vi "CRYO_MASTER_FULL_RUN3.vi"() -> ()   [LabVIEW 2017] (continued)
  in  "CONTROL KIKUSUI?":bool=TRUE
  in  "OUTPUT\n(PWR)":bool
  in  "Set Current (mA)\n (PWR)":dbl=4.0 min=4.0 max=20.0 format="%_3g"
  out "RUN Identifier 5":string="20210209_084357_RUNIII" caption="RUN Identifier"
  in  "DMMsConfig":T11(array[cluster])=[{"Label"="I_H1", "Active?"=TRUE, "VISA resource name"="USB0::0x1334::0x0204::262800066::INSTR", "Device"=enum."ADCMT7351", "Measurement"=enum."DC Currents", "FileFormat"="%.4e"}, {"Label"="V_H1", "Active?"=TRUE, "VISA resource name"="USB0::0x1334::0x0204::262800451::INSTR", "Device"=enum."ADCMT7351", "Measurement"=enum."DC Volts", "FileFormat"="%.4e"}, {"Label"="I_H2", "Active?"=TRUE, "VISA resource name"="GPIB0::23::INSTR", "Device"=enum."ADCMT7451", "Measurement"=enum."DC Currents", "FileFormat"="%.4e"}, {"Label"="V_H2", "Active?"=TRUE, "VISA resource name"="GPIB0::22::INSTR", "Device"=enum."Agilent34401A", "Measurement"=enum."DC Volts", "FileFormat"="%.4e"}, {"Label"="I_H4", "Active?"=TRUE, "VISA resource name"="GPIB0::21::INSTR", "Device"=enum."Agilent34401A", "Measurement"=enum."DC Currents", "FileFormat"="%.4e"}, {"Label"="V_H4", "Active?"=TRUE, "VISA resource name"="GPIB0::25::INSTR", "Device"=enum."Agilent34401A", "Measurement"=enum."DC Volts", "FileFormat"="%.4e"}]
  out "ƒ¢T=T_2 -T_1":dbl=-101388.71309149737
  out "Graph DMMs 3":T4(graph)=[{"TimeArray"=[timestamp(3695672642.6155486 s since 1904-01-01)], "DataArray"=[-2.68e-05]}, {"TimeArray"=[timestamp(3695672642.6155486 s since 1904-01-01)], "DataArray"=[-0.0014684]}, {"TimeArray"=[timestamp(3695672642.6155486 s since 1904-01-01)], "DataArray"=[-1.232e-05]}, {"TimeArray"=[timestamp(3695672642.6155486 s since 1904-01-01)], "DataArray"=[2.8262e-06]}, {"TimeArray"=[timestamp(3695672642.6155486 s since 1904-01-01)], "DataArray"=[3.71392e-06]}, {"TimeArray"=[timestamp(3695672642.6155486 s since 1904-01-01)], "DataArray"=[0.000182]}, {"TimeArray"=[timestamp(3695672642.6155486 s since 1904-01-01)], "DataArray"=[101407.09548804205]}, {"TimeArray"=[timestamp(3695672642.6155486 s since 1904-01-01)], "DataArray"=[-0.36185606613019977]}, {"TimeArray"=[timestamp(3695672642.6155486 s since 1904-01-01)], "DataArray"=[-3.0973798990583647]}, {"TimeArray"=[timestamp(3695672642.6155486 s since 1904-01-01)], "DataArray"=[18.382396544680894]}, {"TimeArray"=[timestamp(3695672642.6155486 s since 1904-01-01)], "DataArray"=[-48.20456535494683]}, {"TimeArray"=[timestamp(3695672642.6155486 s since 1904-01-01)], "DataArray"=[167.919]}, {"TimeArray"=[timestamp(3695672642.6155486 s since 1904-01-01)], "DataArray"=[163.1]}, {"TimeArray"=[timestamp(3695672642.6155486 s since 1904-01-01)], "DataArray"=[162.659]}, {"TimeArray"=[timestamp(3695672642.6155486 s since 1904-01-01)], "DataArray"=[160.848]}] caption="XY Graph"
  out "Q = I *V":dbl=3.935312e-08
  in  "index I":i64
  in  "index V":i64=1
  out "VariableSources":T12(array[ring])=[enum."USB6210", enum."USB6218AI", enum."USB6218AI", enum."USB6218AI", enum."USB6210", enum."LSI336", enum."LSI336", enum."LSI336", enum."LSI336"]
  in  "DMMsConfig (variables)":T13(array[cluster])=[{"Label"="P_3Hepot", "Active?"=TRUE, "Source"=enum."USB6210", "SourceLabel"="P_3Hepot", "FileFormat"="%6.4e"}, {"Label"="F_1", "Active?"=TRUE, "Source"=enum."USB6218AI", "SourceLabel"="F_1", "FileFormat"="%3.4f"}, {"Label"="F_4", "Active?"=TRUE, "Source"=enum."USB6218AI", "SourceLabel"="F_4", "FileFormat"="%3.4f"}, {"Label"="F_5", "Active?"=TRUE, "Source"=enum."USB6218AI", "SourceLabel"="F_5", "FileFormat"="%3.4f"}, {"Label"="DP_HEX4", "Active?"=TRUE, "Source"=enum."USB6210", "SourceLabel"="DP_HEX4", "FileFormat"="%4.3e"}, {"Label"="T3He6-1", "Active?"=TRUE, "Source"=enum."LSI336", "SourceLabel"="T3He6-1", "FileFormat"="%3.4f"}, {"Label"="T3He6-2", "Active?"=TRUE, "Source"=enum."LSI336", "SourceLabel"="T3He6-2", "FileFormat"="%3.4f"}, {"Label"="T3He7-1", "Active?"=TRUE, "Source"=enum."LSI336", "SourceLabel"="T3He7-1", "FileFormat"="%3.4f"}, {"Label"="T3He7-2", "Active?"=TRUE, "Source"=enum."LSI336", "SourceLabel"="T3He7-2", "FileFormat"="%3.4f"}]
  in  "Measure DMMs?":bool=TRUE
  out "DMMsLabels":string[](array[string])=["I_H1", "V_H1", "I_H2", "V_H2", "I_H4", "V_H4", "P_3Hepot", "F_1", "F_4", "F_5", "DP_HEX4", "T3He6-1", "T3He6-2", "T3He7-1", "T3He7-2"]
  out "Active?":bool[](array[boolean])=[TRUE, TRUE, TRUE, TRUE, TRUE, TRUE, TRUE, TRUE, TRUE, TRUE, TRUE, TRUE, TRUE, TRUE, TRUE]
  out "DMM LastMeasurements":dbl[](array[numeric])=[-2.68e-05, -0.0014684, -1.232e-05, 2.8262e-06, 3.71392e-06, 0.000182, 101407.09548804205, -0.36185606613019977, -3.0973798990583647, 18.382396544680894, -48.20456535494683, 167.919, 163.1, 162.659, 160.848]
  out "Graph DMMs 2":T4(graph)=[{"TimeArray"=[timestamp(3695672642.6155486 s since 1904-01-01)], "DataArray"=[-2.68e-05]}, {"TimeArray"=[timestamp(3695672642.6155486 s since 1904-01-01)], "DataArray"=[-0.0014684]}, {"TimeArray"=[timestamp(3695672642.6155486 s since 1904-01-01)], "DataArray"=[-1.232e-05]}, {"TimeArray"=[timestamp(3695672642.6155486 s since 1904-01-01)], "DataArray"=[2.8262e-06]}, {"TimeArray"=[timestamp(3695672642.6155486 s since 1904-01-01)], "DataArray"=[3.71392e-06]}, {"TimeArray"=[timestamp(3695672642.6155486 s since 1904-01-01)], "DataArray"=[0.000182]}, {"TimeArray"=[timestamp(3695672642.6155486 s since 1904-01-01)], "DataArray"=[101407.09548804205]}, {"TimeArray"=[timestamp(3695672642.6155486 s since 1904-01-01)], "DataArray"=[-0.36185606613019977]}, {"TimeArray"=[timestamp(3695672642.6155486 s since 1904-01-01)], "DataArray"=[-3.0973798990583647]}, {"TimeArray"=[timestamp(3695672642.6155486 s since 1904-01-01)], "DataArray"=[18.382396544680894]}, {"TimeArray"=[timestamp(3695672642.6155486 s since 1904-01-01)], "DataArray"=[-48.20456535494683]}, {"TimeArray"=[timestamp(3695672642.6155486 s since 1904-01-01)], "DataArray"=[167.919]}, {"TimeArray"=[timestamp(3695672642.6155486 s since 1904-01-01)], "DataArray"=[163.1]}, {"TimeArray"=[timestamp(3695672642.6155486 s since 1904-01-01)], "DataArray"=[162.659]}, {"TimeArray"=[timestamp(3695672642.6155486 s since 1904-01-01)], "DataArray"=[160.848]}] caption="XY Graph"
  out "DMMFileName":string="20210209_084357_RUNIII_DMMs_20210209_084357.csv"
  out "error out (DMMs)":errorcluster
  out "cycle # (DMMs)":i32=1
  in  "Measurement Interval DMMs (ms)":i64=500
  in  "InstName DMMs":string="DMMs"
  in  "Initialize (DMMs)":bool
  out "Graph DMMs 1":T4(graph)=[{"TimeArray"=[timestamp(3695672642.6155486 s since 1904-01-01)], "DataArray"=[-2.68e-05]}, {"TimeArray"=[timestamp(3695672642.6155486 s since 1904-01-01)], "DataArray"=[-0.0014684]}, {"TimeArray"=[timestamp(3695672642.6155486 s since 1904-01-01)], "DataArray"=[-1.232e-05]}, {"TimeArray"=[timestamp(3695672642.6155486 s since 1904-01-01)], "DataArray"=[2.8262e-06]}, {"TimeArray"=[timestamp(3695672642.6155486 s since 1904-01-01)], "DataArray"=[3.71392e-06]}, {"TimeArray"=[timestamp(3695672642.6155486 s since 1904-01-01)], "DataArray"=[0.000182]}, {"TimeArray"=[timestamp(3695672642.6155486 s since 1904-01-01)], "DataArray"=[101407.09548804205]}, {"TimeArray"=[timestamp(3695672642.6155486 s since 1904-01-01)], "DataArray"=[-0.36185606613019977]}, {"TimeArray"=[timestamp(3695672642.6155486 s since 1904-01-01)], "DataArray"=[-3.0973798990583647]}, {"TimeArray"=[timestamp(3695672642.6155486 s since 1904-01-01)], "DataArray"=[18.382396544680894]}, {"TimeArray"=[timestamp(3695672642.6155486 s since 1904-01-01)], "DataArray"=[-48.20456535494683]}, {"TimeArray"=[timestamp(3695672642.6155486 s since 1904-01-01)], "DataArray"=[167.919]}, {"TimeArray"=[timestamp(3695672642.6155486 s since 1904-01-01)], "DataArray"=[163.1]}, {"TimeArray"=[timestamp(3695672642.6155486 s since 1904-01-01)], "DataArray"=[162.659]}, {"TimeArray"=[timestamp(3695672642.6155486 s since 1904-01-01)], "DataArray"=[160.848]}] caption="XY Graph"
  out "error out (DMM graphs)":errorcluster
  in  "Sample #":i32=5
  in  "index T_ 1":i64=6
  in  "index T_2":i64=9
  out "error out (DMMs) 2":errorcluster
  out "P_HEX7OUT":dbl=101021.4665932051 format="%_4e"
  out "P (HEX7 out)":dbl=101021.4665932051 format="%_4e"
  out "DP HEX5":dbl=-4.397643774686294 format="%_4e"
  out "DP_HEX5":dbl=-4.397643774686294 format="%_4e"
  in  "Diff pressure HEX5":string="DP_HEX5"
  out "3He pot level":dbl=7.365405585846229 format="%_4f"
  in  "3He pot":string="L1"
  out "He level (3He)":dbl(slide)=7.365405585846229 scale=0.0..100.0
  out "He level (1K) b":dbl(slide)=-0.047872817403439266 scale=0.0..100.0
  out "He level (1K)":dbl(slide)=0.13428935722636412 scale=0.0..100.0
  out "He level (4K)":dbl(slide)=-0.023540685641880416 scale=0.0..100.0
  out "1K pot(b1)":dbl=-0.047872817403439266 format="%_4f"
  in  "1K pot (b)":string="L2-2"
  in  "1K pot level":string="L2-1"
  out "L(1K) (a1)":dbl=0.13428935722636412 format="%_4f"
  in  "SensorLocation 2":T14(ring)=enum."T3He5"
  out "Temperature 2":dbl=167.912
  out "DP HEX4":dbl=-47.57146989712546 format="%_4e"
  in  "Diff pressure HEX4":string="DP_HEX4"
  out "V2":bool
  out "V1":bool=TRUE
  out "F5 (1K pump ex.)":dbl=17.202044578830606 format="%_4f"
  out "F4 (3He in to HEX7)":dbl=-7.769469766427424 format="%_3f"
  out "F3 (4He rtn flw via HEX7)":dbl=2.98269711881182 format="%_4f"
  out "F1 (3He pump exhaust) flow":dbl=-5.195052785009831 format="%_4f"
  out "P (Dewar)":dbl=102950.69349153554 format="%_4e"
  out "P (1K pot)":dbl=101443.04292994068 format="%_4e"
  out "P (3He pot)":dbl=101551.76197190638 format="%_4e"
  out "P (shield return)":dbl=101480.26148830613 format="%_4e"
  out "P (3He IN)":dbl=100240.36414180837 format="%_4e"
  out "P (4K reservoir)":dbl=97813.1918911886 format="%_4e"
  out "P (insulation)":dbl=18.32747458588863 format="%_4e"
  in  "1Kpot pump exhaust flow":string="F_5"
  out "F_5":dbl=17.202044578830606 format="%_4f"
  in  "3He incoming flow into HEX7":string="F_4"
  out "F_4":dbl=-7.769469766427424 format="%_4f"
  out "F_3":dbl=2.98269711881182 format="%_4f"
  in  "4He return flow from HEX7":string="F_3"
  out "F_2":dbl=0.20377377393752083 format="%_4f"
  in  "Shield flow":string="F_2"
  out "P_SldRTN":dbl=101480.26148830613 format="%_4e"
  in  "3He pot pressure":string="P_3Hepot"
  out "P_3Hepot":dbl=101551.76197190638 format="%_4e"
  in  "Shield return press.":string="P_SldRTN"
  out "F_1":dbl=-5.195052785009831 format="%_4f"
  in  "3He pump exhaust flow":string="F_1"
  out "P_Dewar":dbl=102950.69349153554 format="%_4e"
  in  "Dewar pressure":string="P_Dewar"
  out "P_1Kpot":dbl=101443.04292994068 format="%_4e"
  in  "1Kpot pressure":string="P_1Kpot"
  out "P_3HeIN":dbl=100240.36414180837 format="%_4e"
  in  "3He inlet pressure":string="P_3HeIN"
  in  "4K reservoir pressure":string="P_4Kres"
  out "P_4Kres":dbl=97813.1918911886 format="%_4e"
  out "P_ins":dbl=18.32747458588863 format="%_4e"
  in  "Insulation vacuum":string="P_ins"
  out "T3He7-1/6-2 (3He pot) 2":dbl=159.065 format="%_4f"
  out "T3He7-1/7-2 (HEX1)":dbl=160.911 format="%_4f"
  out "T3He6-1/6-2 (3He pot) 2":dbl=161.329 format="%_4f"
  out "T3He6-1/6-2 (HEX1)":dbl=166.258 format="%_4f"
  out "T1K3-1/3-2 (1K pot) 2":dbl=116.203 format="%_4f"
  out "T1K3-1/3-2 (1K pot)":dbl=116.239 format="%_4f"
  out "T4He1 (4K reservoir )":dbl=127.38 format="%_4f"
  out "Temperature 1":dbl=206.95
  in  "SensorLocation 1":T14(ring)=enum."TTH2"
  out "TIP7":dbl format="%_4g"
  out "T3He6-2":dbl=161.329 format="%_4g"
  out "T3He7-2":dbl=159.065 format="%_4g"
  out "T3He6-1":dbl=166.258 format="%_4g"
  out "T3He4":dbl=154.09 format="%_4g"
  out "T3He7-1":dbl=160.911 format="%_4g"
  out "T3He8":dbl=127.318 format="%_4g"
  out "T3He5":dbl=167.912 format="%_4g"
  out "T1K3-2":dbl=116.203 format="%_4g"
  out "T1K3-1":dbl=116.239 format="%_4g"
  out "TIP6":dbl=147.89 format="%_4g"
  out "T3He9":dbl=137.88 format="%_4g"
  out "T1K5":dbl=143.12 format="%_4g"
  out "T1K4":dbl=127.59 format="%_4g"
  out "T1K2":dbl=178.09 format="%_4g"
  out "TIP5":dbl=172.64 format="%_4g"
  out "TIP4":dbl=147.93 format="%_4g"
  out "TIP3":dbl=215.82 format="%_4g"
  out "TIP2":dbl=231.74 format="%_4g"
  out "TIP1":dbl=279.25 format="%_4g"
  out "T1K6":dbl=286.82 format="%_4g"
  out "T4He10":dbl=274.41 format="%_4g"
  out "T4He8":dbl=281.47 format="%_4g"
  out "T4He7":dbl=256.33 format="%_4g"
  out "T3He1-3":dbl=289.96 format="%_4g"
  out "T3He1-2":dbl=292.25 format="%_4g"
  out "T4He9":dbl=226.25 format="%_4g"
  out "T4He6":dbl=213.01 format="%_4g"
  out "T4He5":dbl=217.43 format="%_4g"
  out "T4He4":dbl=214.31 format="%_4g"
  out "T4He2-2":dbl=204.35 format="%_4g"
  out "T4He2-1":dbl=215.52 format="%_4g"
  out "T4He3-4":dbl=290.83 format="%_4g"
  out "T4He3-3":dbl=290.77 format="%_4g"
  out "T4He3-2":dbl=292.95 format="%_4g"
  out "T4He3-1":dbl=292.82 format="%_4g"
  out "T3He1-4":dbl=289.7 format="%_4g"
  out "T3He3":dbl=159.56 format="%_4g"
  out "T3He2-2":dbl=208.05 format="%_4g"
  out "T3He2-1":dbl=213.16 format="%_4g"
  out "T1K1":dbl=156.15 format="%_4g"
  out "T4He1":dbl=127.38 format="%_4g"
  out "TTH1":dbl=191.48 format="%_4g"
  out "TTH2":dbl=206.95 format="%_4g"
  out "TTH4":dbl=242.22 format="%_4g"
  out "TTH3":dbl=244.99 format="%_4g"
  out "T3He1-1":dbl=291.98 format="%_4g"
  out "T3He10":dbl=285.72 format="%_4g"
  out "F2 (shield flow)":dbl=0.20377377393752083 format="%_4f"
  out "DP_HEX4":dbl=-47.57146989712546 format="%_4e"
  in  "4K reservoir level":string="L3"
  out "L3":dbl=-0.023540685641880416 format="%_4f"
  out "RUN Identifier 6":string="20210209_084357_RUNIII" caption="RUN Identifier"
  in  "HEX7 out pressure":string="P_HEX7OUT"
  in  "STOP CHF":bool
  in  "CHF Graph Comment":string="CHF_TEST2"
  in  "REFRESH GRAPH":bool
  in  "RECORD GRAPH":bool
  out "Graph CHF log 2":T4(graph) caption="XY Graph"
  out "ƒ¢T_array":dbl[](array[numeric])=[52.7753, 52.7753, 52.7113, 52.7149, 52.7149, 52.4737, 52.4737, 52.4737, 52.3482, 52.3482, 52.178799999999995, 52.165000000000006, 52.165000000000006, 52.165000000000006, 52.0492, 52.0492, 51.9912, 51.9912, 51.9912, 51.7804, 51.7804, 51.7804, 51.6556, 51.6556, 51.6556, 51.5194, 51.5194, 51.447500000000005, 51.3779, 51.3779, 51.3779, 51.1899, 51.1899, 51.2118, 51.2118, 51.2118, 51.182199999999995, 51.1555, 51.1555, 51.0157, 51.0157, 51.0157, 50.9915, 50.9915, 50.8838, 50.926899999999996, 50.926899999999996, 50.861599999999996, 50.861599999999996, 50.861599999999996, 50.876400000000004, 50.876400000000004, 50.748400000000004, 50.7998, 50.7998, 50.7998, 50.7818, 50.7818, 50.8097, 50.8097, 50.8097, 50.7905, 50.7905, 50.7905, 50.8299, 50.8299, 50.8299, 50.8304, 50.8304, 50.8908, 50.884699999999995, 50.884699999999995, 51.0378, 51.0378, 51.0378, 51.019000000000005, 51.019000000000005, 51.120799999999996, 51.156600000000005, 51.156600000000005, 51.156600000000005, 51.2329, 51.2329, 51.369299999999996, 51.369299999999996, 51.369299999999996, 51.5356, 51.5356, 51.5356, 51.6671, 51.6671, 51.6671, 51.8208, 51.8208, 51.987899999999996, 52.0073, 52.0073, 52.2344, 52.2344, 52.2344, 52.459, 52.459, 52.672399999999996, 52.708999999999996, 52.708999999999996, 52.708999999999996, 52.9287, 52.9287, 53.1942, 53.1942, 53.1942, 53.5324, 53.5324, 53.5324, 53.849000000000004, 53.849000000000004, 53.849000000000004, 54.1092, 54.1092, 54.4229, 54.5156, 54.5156, 54.8154, 54.8154, 54.8154, 55.2085, 55.2085, 55.5868, 55.656800000000004, 55.656800000000004]
  out "Graph CHF":cluster{dbl[], dbl[]}(graph)={[52.7753, 52.7753, 52.7113, 52.7149, 52.7149, 52.4737, 52.4737, 52.4737, 52.3482, 52.3482, 52.178799999999995, 52.165000000000006, 52.165000000000006, 52.165000000000006, 52.0492, 52.0492, 51.9912, 51.9912, 51.9912, 51.7804, 51.7804, 51.7804, 51.6556, 51.6556, 51.6556, 51.5194, 51.5194, 51.447500000000005, 51.3779, 51.3779, 51.3779, 51.1899, 51.1899, 51.2118, 51.2118, 51.2118, 51.182199999999995, 51.1555, 51.1555, 51.0157, 51.0157, 51.0157, 50.9915, 50.9915, 50.8838, 50.926899999999996, 50.926899999999996, 50.861599999999996, 50.861599999999996, 50.861599999999996, 50.876400000000004, 50.876400000000004, 50.748400000000004, 50.7998, 50.7998, 50.7998, 50.7818, 50.7818, 50.8097, 50.8097, 50.8097, 50.7905, 50.7905, 50.7905, 50.8299, 50.8299, 50.8299, 50.8304, 50.8304, 50.8908, 50.884699999999995, 50.884699999999995, 51.0378, 51.0378, 51.0378, 51.019000000000005, 51.019000000000005, 51.120799999999996, 51.156600000000005, 51.156600000000005, 51.156600000000005, 51.2329, 51.2329, 51.369299999999996, 51.369299999999996, 51.369299999999996, 51.5356, 51.5356, 51.5356, 51.6671, 51.6671, 51.6671, 51.8208, 51.8208, 51.987899999999996, 52.0073, 52.0073, 52.2344, 52.2344, 52.2344, 52.459, 52.459, 52.672399999999996, 52.708999999999996, 52.708999999999996, 52.708999999999996, 52.9287, 52.9287, 53.1942, 53.1942, 53.1942, 53.5324, 53.5324, 53.5324, 53.849000000000004, 53.849000000000004, 53.849000000000004, 54.1092, 54.1092, 54.4229, 54.5156, 54.5156, 54.8154, 54.8154, 54.8154, 55.2085, 55.2085, 55.5868, 55.656800000000004, 55.656800000000004], [64.988847618, 0.0008371808639999999, 0.0008371808639999999, 0.0008371808639999999, 0.0008371808639999999, 0.0008371808639999999, 0.0008371808639999999, 0.0008371808639999999, 0.0008371808639999999, 0.0008371808639999999, 0.027133083646800005, 0.027133083646800005, 0.027133083646800005, 0.027133083646800005, 0.027133083646800005, 0.027133083646800005, 0.027133083646800005, 0.027133083646800005, 0.497141592024, 0.497141592024, 0.497141592024, 0.497141592024, 0.497141592024, 0.497141592024, 0.497141592024, 0.497141592024, 1.476215545728, 1.476215545728, 1.476215545728, 1.476215545728, 1.476215545728, 1.476215545728, 1.476215545728, 1.476215545728, 1.476215545728, 3.02773055424, 3.02773055424, 3.02773055424, 3.02773055424, 3.02773055424, 3.02773055424, 3.02773055424, 3.02773055424, 4.86484683444, 4.86484683444, 4.86484683444, 4.86484683444, 4.86484683444, 4.86484683444, 4.86484683444, 4.86484683444, 4.86484683444, 7.4475440352, 7.4475440352, 7.4475440352, 7.4475440352, 7.4475440352, 7.4475440352, 7.4475440352, 7.4475440352, 10.986195312400001, 10.986195312400001, 10.986195312400001, 10.986195312400001, 10.986195312400001, 10.986195312400001, 10.986195312400001, 10.986195312400001, 14.5582761144, 14.5582761144, 14.5582761144, 14.5582761144, 14.5582761144, 14.5582761144, 14.5582761144, 14.5582761144, 14.5582761144, 16.831454674799996, 16.831454674799996, 16.831454674799996, 16.831454674799996, 16.831454674799996, 16.831454674799996, 16.831454674799996, 16.831454674799996, 23.431170976799997, 23.431170976799997, 23.431170976799997, 23.431170976799997, 23.431170976799997, 23.431170976799997, 23.431170976799997, 23.431170976799997, 28.729140804, 28.729140804, 28.729140804, 28.729140804, 28.729140804, 28.729140804, 28.729140804, 28.729140804, 28.729140804, 31.9837009252, 31.9837009252, 31.9837009252, 31.9837009252, 31.9837009252, 31.9837009252, 31.9837009252, 31.9837009252, 40.691919848000005, 40.691919848000005, 40.691919848000005, 40.691919848000005, 40.691919848000005, 40.691919848000005, 40.691919848000005, 40.691919848000005, 47.4670420756, 47.4670420756, 47.4670420756, 47.4670420756, 47.4670420756, 47.4670420756, 47.4670420756, 47.4670420756, 47.4670420756, 50.1891742, 50.1891742, 50.1891742]}
  in  "V_lim_low (V)":dbl format="%_5f"
  in  "V_lim_up (V)":dbl=120.0 format="%_5f"
  out "V":dbl=52.931
  out "I":dbl=0.9481999999999999
  out "Q":dbl=50.1891742
  out "T_low":dbl=4.3544
  out "CHF log file name":string="20210205_150936_RUNIII_20210205_155058_CHFlog.csv"
  in  "Data T_low":T15={"Source"=enum."LSI336", "SourceLabel"="T3He6-1"}
  in  "Data T_high":T15={"Source"=enum."LSI336", "SourceLabel"="T3He7-2"}
  in  "RecordSettings":T16(array[cluster])=[{"Source"=enum."DMMs", "SourceLabel"="I_H1", "FileFormat"="%4.4e"}, {"Source"=enum."DMMs", "SourceLabel"="V_H1", "FileFormat"="%4.4f"}, {"Source"=enum."USB6210", "SourceLabel"="P_3Hepot", "FileFormat"="%4.4e"}, {"Source"=enum."USB6218AI", "SourceLabel"="F_1", "FileFormat"="%4.4f"}, {"Source"=enum."USB6218AI", "SourceLabel"="F_4", "FileFormat"="%4.4f"}, {"Source"=enum."USB6218AI", "SourceLabel"="F_5", "FileFormat"="%4.4f"}, {"Source"=enum."USB6210", "SourceLabel"="DP_HEX4", "FileFormat"="%4.4e"}, {"Source"=enum."LSI336", "SourceLabel"="T3He6-1", "FileFormat"="%4.4f"}, {"Source"=enum."LSI336", "SourceLabel"="T3He6-2", "FileFormat"="%4.4f"}, {"Source"=enum."LSI336", "SourceLabel"="T3He7-1", "FileFormat"="%4.4f"}, {"Source"=enum."LSI336", "SourceLabel"="T3He7-2", "FileFormat"="%4.4f"}, {"Source"=enum."LSI336", "SourceLabel"="T1K3-1", "FileFormat"="%4.4f"}, {"Source"=enum."LSI336", "SourceLabel"="T1K3-2", "FileFormat"="%4.4f"}]
  in  "Data V":T15={"Source"=enum."DMMs", "SourceLabel"="V_H1"}
  in  "Data I":T15={"Source"=enum."DMMs", "SourceLabel"="I_H1"}
  in  "START CHF":bool
  in  "CHF cycle interval (s) (>1s)":dbl=1.0 format="%_3f"
  in  "V_end (V)":dbl=65.0 format="%_4f"
  in  "V start (V)":dbl format="%_4f"
  in  "ƒ¢V / cycle (V)":dbl=0.5 format="%_4f"
  out "error out (Agilent)":errorcluster
  in  "VISA (Agilent 34402)":refnum<visa-resource-name>="USB0::0x0957::0x0407::MY44010230::INSTR"
  out "Agilent\nIntialized?":bool
  in  "Initialize (Agilent)":bool=TRUE
  in  "OUTPUT \nKenwood":bool
  in  "Kenwood set V (V)":dbl min=0.0 max=120.0 format="%_5f"
  out "Graph CHF log 1":T4(graph) caption="XY Graph"
  out "CHF Data Labels":string[](array[string])=["I_H1", "V_H1", "P_3Hepot", "F_1", "F_4", "F_5", "DP_HEX4", "T3He6-1", "T3He6-2", "T3He7-1", "T3He7-2", "T1K3-1", "T1K3-2"]
  out "CHF last data":dbl[](array[numeric])=[0.9481999999999999, 52.931, 102652.98108709365, 62.055409553750465, -0.5229626466829013, 2.2553033880524875, -50.30940195270617, 4.3544, 51.4202, 48.6656, 60.0112, 4.2108, 4.2278]
  out "Error out (CHF rec)":errorcluster
  out "CHF measurement counter":i32
  out "T_high":dbl=60.0112
  out "ƒ¢T":dbl=55.656800000000004
  out "Q_array":dbl[](array[numeric])=[64.988847618, 0.0008371808639999999, 0.0008371808639999999, 0.0008371808639999999, 0.0008371808639999999, 0.0008371808639999999, 0.0008371808639999999, 0.0008371808639999999, 0.0008371808639999999, 0.0008371808639999999, 0.027133083646800005, 0.027133083646800005, 0.027133083646800005, 0.027133083646800005, 0.027133083646800005, 0.027133083646800005, 0.027133083646800005, 0.027133083646800005, 0.497141592024, 0.497141592024, 0.497141592024, 0.497141592024, 0.497141592024, 0.497141592024, 0.497141592024, 0.497141592024, 1.476215545728, 1.476215545728, 1.476215545728, 1.476215545728, 1.476215545728, 1.476215545728, 1.476215545728, 1.476215545728, 1.476215545728, 3.02773055424, 3.02773055424, 3.02773055424, 3.02773055424, 3.02773055424, 3.02773055424, 3.02773055424, 3.02773055424, 4.86484683444, 4.86484683444, 4.86484683444, 4.86484683444, 4.86484683444, 4.86484683444, 4.86484683444, 4.86484683444, 4.86484683444, 7.4475440352, 7.4475440352, 7.4475440352, 7.4475440352, 7.4475440352, 7.4475440352, 7.4475440352, 7.4475440352, 10.986195312400001, 10.986195312400001, 10.986195312400001, 10.986195312400001, 10.986195312400001, 10.986195312400001, 10.986195312400001, 10.986195312400001, 14.5582761144, 14.5582761144, 14.5582761144, 14.5582761144, 14.5582761144, 14.5582761144, 14.5582761144, 14.5582761144, 14.5582761144, 16.831454674799996, 16.831454674799996, 16.831454674799996, 16.831454674799996, 16.831454674799996, 16.831454674799996, 16.831454674799996, 16.831454674799996, 23.431170976799997, 23.431170976799997, 23.431170976799997, 23.431170976799997, 23.431170976799997, 23.431170976799997, 23.431170976799997, 23.431170976799997, 28.729140804, 28.729140804, 28.729140804, 28.729140804, 28.729140804, 28.729140804, 28.729140804, 28.729140804, 28.729140804, 31.9837009252, 31.9837009252, 31.9837009252, 31.9837009252, 31.9837009252, 31.9837009252, 31.9837009252, 31.9837009252, 40.691919848000005, 40.691919848000005, 40.691919848000005, 40.691919848000005, 40.691919848000005, 40.691919848000005, 40.691919848000005, 40.691919848000005, 47.4670420756, 47.4670420756, 47.4670420756, 47.4670420756, 47.4670420756, 47.4670420756, 47.4670420756, 47.4670420756, 47.4670420756, 50.1891742, 50.1891742, 50.1891742]
  out "CHF file name":string="20210205_150936_RUNIII_CHF20210205_154539_CHF_TEST1.csv"
  out "Graph CHF log 3":T4(graph) caption="XY Graph"
  out "File Refnum (CHF)":refnum<file>
  out "Series 1":string[](array[string])=["P_ins", "P_4Kres", "P_3HeIN", "P_SldRTN", "P_3Hepot", "P_1Kpot", "P_Dewar(old)", "P_HEX7OUT", "P_IP", "P_Dewar"]
  out "Series 2":string[](array[string])=["DP_HEX4", "DP_HEX5", "L1(old)", "L2-1", "L2-2", "L3", "R_L1", "L1"]
  out "Series 3":string[](array[string])=["F_1", "F_2", "F_3", "F_4", "F_5", "I_CV"]
  out "Series 4":string[](array[string])=["TTH3", "TTH4", "TTH1", "TTH2", "T4He1", "T1K1", "T3He2-1", "T3He2-2", "T4He3-1", "T4He3-2", "T4He3-3", "T4He3-4", "T4He2-1", "T4He2-2", "T4He4", "T1K2", "T1K4", "T1K5", "T3He4", "T1K3-1", "T1K3-2", "T3He5", "T3He8", "T3He6-1", "T3He6-2", "T3He7-1", "T3He7-2"]
  out "Plot errors":errorcluster
  out "LastMeasurementConfig (218)":T17(array[cluster])=[{"LSIName"="LSI218A", "Active?"=TRUE, "LastData"=[286.39, 292.79, 245.71, 242.82, 192.73, 208.05, 129.14, 157.86], "Labels"=["T3He10", "T3He1-1", "TTH3", "TTH4", "TTH1", "TTH2", "T4He1", "T1K1"]}, {"LSIName"="LSI218B", "Active?"=TRUE, "LastData"=[30.0, 0.0, 0.0, 0.0, 214.32, 209.26, 161.19, 290.41], "Labels"=["N.C.", "N.C.", "N.C.", "N.C.", "T3He2-1", "T3He2-2", "T3He3", "T3He1-4"]}, {"LSIName"="LSI218C", "Active?"=TRUE, "LastData"=[293.53, 293.65, 291.53, 291.58, 216.58, 205.59, 215.41, 218.49], "Labels"=["T4He3-1", "T4He3-2", "T4He3-3", "T4He3-4", "T4He2-1", "T4He2-2", "T4He4", "T4He5"]}, {"LSIName"="LSI218D", "Active?"=TRUE, "LastData"=[214.17, 227.11, 292.96, 290.69, 256.79, 281.72, 274.72, 287.38], "Labels"=["T4He6", "T4He9", "T3He1-2", "T3He1-3", "T4He7", "T4He8", "T4He10", "T1K6"]}, {"LSIName"="LSI218E", "Active?"=TRUE, "LastData"=[279.49, 0.0, 232.53, 688.49, 216.83, 149.55, 173.98, 688.58], "Labels"=["TIP1", "N.C.", "TIP2", "N.C.", "TIP3", "TIP4", "TIP5", "N.C."]}, {"LSIName"="LSI218F", "Active?"=TRUE, "LastData"=[178.46, 128.79, 144.74, 152.95, 140.88, 150.1, 0.433, 0.0], "Labels"=["T1K2", "T1K4", "T1K5", "T3He4", "T3He9", "TIP6", "N.C.", "N.C."]}]
  out "DataArrayConv (USB6210)":dbl[][](array[numeric])=[[18.674861858538797, 97865.81349287118, 100998.44453584745, 100709.02551899779, 101407.09548804205, 101279.08758660906, 0.0, -48.20456535494683, 0.06691412080322978, 10.108489682314854, 0.1698011167381339, -0.07483544992953703, 0.04024895650740204, 100273.25274306418, 4.684755546764993e-05, 5.953981760223165]]
  out "LastMeasurementConfig (336)":T17(array[cluster])=[{"LSIName"="LSi336X", "Active?"=TRUE, "LastData"=[117.963, 117.927, 169.419, 129.275], "Labels"=["T1K3-1", "T1K3-2", "T3He5", "T3He8"]}, {"LSIName"="LSi336Y", "Active?"=TRUE, "LastData"=[167.919, 163.1, 162.659, 160.848], "Labels"=["T3He6-1", "T3He6-2", "T3He7-1", "T3He7-2"]}]
  out "DataArrayConv (USB6218)":dbl[][](array[numeric])=[[-0.36185606613019977, -1.4204433335631088, 0.28794373208354185, -3.0973798990583647, 18.382396544680894, -0.0024966396874153696, -25.07402456902091, 102243.79868545999, 107.20664477077275]]
  out "TimeArray (USB6218)":timestamp[](array[timestamp])=[timestamp(3695672639.4136896 s since 1904-01-01)]
  out "Data Array sizes (6210)":i32[](array[numeric])=[1, 16]
  out "DataArraySize (6218)":i32[](array[numeric])=[1, 9]
  out "TimeArray size (6218)":i32=1
  out "TimeArray (LSI336)":timestamp[](array[timestamp])=[timestamp(3695672639.4087214 s since 1904-01-01)]
  out "TimeArray Size (336)":i32=1
  out "DataArray (336)":dbl[][](array[numeric])=[[117.963, 117.927, 169.419, 129.275, 167.919, 163.1, 162.659, 160.848]]
  out "DataArray size (336)":i32[](array[numeric])=[1, 8]
  out "LastData (LSI218)":dbl[](array[numeric])=[286.39, 292.79, 245.71, 242.82, 192.73, 208.05, 129.14, 157.86, 30.0, 0.0, 0.0, 0.0, 214.32, 209.26, 161.19, 290.41, 293.53, 293.65, 291.53, 291.58, 216.58, 205.59, 215.41, 218.49, 214.17, 227.11, 292.96, 290.69, 256.79, 281.72, 274.72, 287.38, 279.49, 0.0, 232.53, 688.49, 216.83, 149.55, 173.98, 688.58, 178.46, 128.79, 144.74, 152.95, 140.88, 150.1, 0.433, 0.0]
  out "TempSensorsLocations":T18(array[ring])=[enum."T3He10", enum."T3He1-1", enum."TTH3", enum."TTH4", enum."TTH1", enum."TTH2", enum."T4He1", enum."T1K1", enum."N.C.", enum."N.C.", enum."N.C.", enum."N.C.", enum."T3He2-1", enum."T3He2-2", enum."T3He3", enum."T3He1-4", enum."T4He3-1", enum."T4He3-2", enum."T4He3-3", enum."T4He3-4", enum."T4He2-1", enum."T4He2-2", enum."T4He4", enum."T4He5", enum."T4He6", enum."T4He9", enum."T3He1-2", enum."T3He1-3", enum."T4He7", enum."T4He8", enum."T4He10", enum."T1K6", enum."TIP1", enum."N.C.", enum."TIP2", enum."N.C.", enum."TIP3", enum."TIP4", enum."TIP5", enum."N.C.", enum."T1K2", enum."T1K4", enum."T1K5", enum."T3He4", enum."T3He9", enum."TIP6", enum."N.C.", enum."N.C.", enum."T1K3-1", enum."T1K3-2", enum."T3He5", enum."T3He8", enum."T3He6-1", enum."T3He6-2", enum."T3He7-1", enum."T3He7-2"]
  out "AllTemperatures":dbl[](array[numeric])=[285.72, 291.98, 244.99, 242.22, 191.48, 206.95, 127.38, 156.15, 30.0, 0.0, 0.0, 0.0, 213.16, 208.05, 159.56, 289.7, 292.82, 292.95, 290.77, 290.83, 215.52, 204.35, 214.31, 217.43, 213.01, 226.25, 292.25, 289.96, 256.33, 281.47, 274.41, 286.82, 279.25, 0.0, 231.74, 688.49, 215.82, 147.93, 172.64, 688.58, 178.09, 127.59, 143.12, 154.09, 137.88, 147.89, 0.433, 0.0, 116.239, 116.203, 167.912, 127.318, 166.258, 161.329, 160.911, 159.065]
  out "error out (frontpanel screenshots)":errorcluster
  out "error out (graph operations)":errorcluster
  out "error out (monthly folder creation)":errorcluster={"status"=TRUE, "code"=10, "source"="Create Folder in CRYO_MASTER_FULL_RUN3.vi<APPEND>\nC:\\LabVIEW\\DATA\\Google\\TUCAN Experiments\\KEK_cryotests_2019-2020\\data\\screenshots\\202102"}
  out "RUN Identifier 7":string="20210209_084357_RUNIII" caption="RUN Identifier"
  out "error out (notifier)":errorcluster
  # "GLOBAL STATUS/CONTROL"
  # "Global Settings"
  # "USB6210 Analog inputs Settings"
  # "USB6218 Analog inputs Settings"
  # "USB6218 Digital Output Settings"
  # "USB6218 Analog Output Settings"
  # "LSI218 Settings"
  # "LSI336 Settings"
  # "HP 34401A (He level meter)"
  # "Graph screenshots"
  # "Configuration"
  # "Activated only when *FIll state* = TRUE"
  # "Activated only when *FIll state* = TRUE"
  # "Vavle Status"
  # "OPEN"
  # "CLOSED"
  # "ADCMT6240A Control/Status"
  # "ADCMT6240A Initialization"
  # "Set Currents (mA)"
  # "PWR400H CTRL via USB6218"
  # "PMC18-3A CTRL via USB621"
  # "DMM configurations"
  # "DMM measurements"
  # "CAUTION: ADCMT 7351 does not have 4-wire resistance measurement function. \n 4-Wire Resistance --> 2-Wire Resistance wih Low Power for this device"
  # "Representative temperatures"
  # "Pressures / Flows"
  # "Labels"
  # "Values"
  # "Helium Levels"
  # "Manual Control of Kenwood"
  # "Automatic Measurement"
  # "Before the measurement\n - Intialize Agilent 34402 (FG)\n - Refresh the CHF graph if necessary\n - Go to DMMs tab and check that DMM measurement is running \n - Fill in the CHF measurement parameters below \nThen press START CHF!"
  # "Measurement Configurations"
  # "Channel selection"
  # "Q = I x V"
  # "ƒ¢T = T_high - T_low"
  # "Record Configurations"
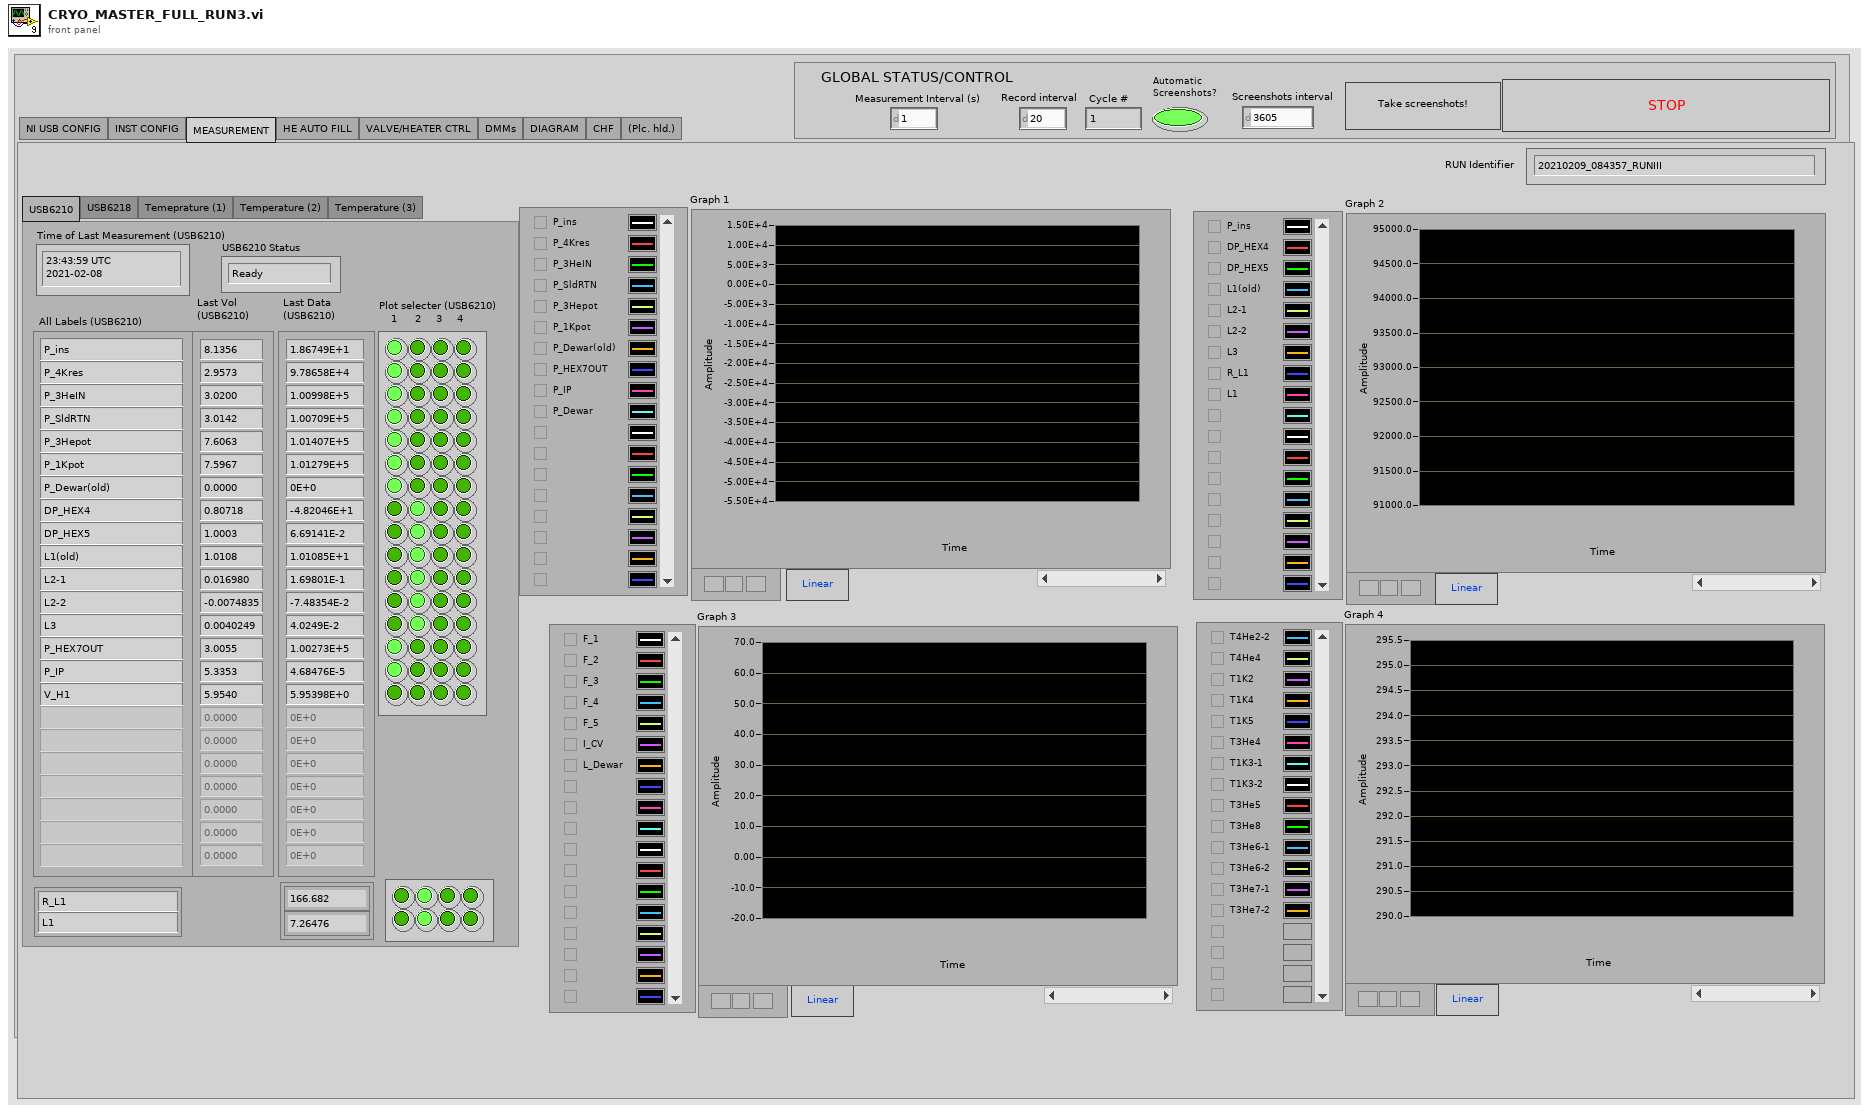
[diagram p1: front panel]
types:
  T1 = enum32{"NI USB CONFIG", "INST CONFIG", "MEASUREMENT", "HE AUTO FILL", "VALVE/HEATER CTRL", "DMMs", "DIAGRAM", "CHF", "(Plc. hld.)"}
  T2 = cluster{"Label":string, "FileFormat":string, "Active?":bool, "Physical CH":tag, " terminal\n type":i32, "ConversionType":cluster{"Type":enum16{"Raw", "SimpleProp", "CC-10_COMBINED", "CC-10_LOG", "LeakDet_EXP", "LeakDet_Mantissa", "Baratron"}, "ConversionParameters":dbl[]}, "VoltageLimits":dbl[]}[]
  T3 = cluster{"LSIName":string, "Labels":string[], "SensorLocations":enum16{"N.C.", "T3He1-1", "T3He1-2", "T3He1-3", "T3He1-4", "T3He2-1", "T3He2-2", "T3He3", "T3He4", "T3He5", "T3He6-1", "T3He6-2", "T3He7-1", "T3He7-2", "T3He8", "T3He9", "T3He10", "T4He1", "T4He2-1", "T4He2-2", "T4He3-1", "T4He3-2", "T4He3-3", "T4He3-4", "T4He4", "T4He5", "T4He6", "T4He7", "T4He8", "T4He9", "T4He10", "T1K1", "T1K2", "T1K3-1", "T1K3-2", "T1K4", "T1K5", "T1K6", "TIP1", "TIP2", "TIP3", "TIP4", "TIP5", "TIP6", "TIP7", "TTH1", "TTH2", "TTH3", "TTH4"}[], "Active?":bool, "VISA res. name":refnum<visa-resource-name>}[]
  T4 = cluster{"TimeArray":timestamp[], "DataArray":dbl[]}[]
  T5 = enum32{"USB6210", "USB6218", "Temeprature (1)", "Temperature (2)", "Temperature (3)"}
  T6 = enum16{"Intialized", "Ready", "Measuring", "Terminated"}
  T7 = enum16{"Initialized", "Ready", "Measuring", "Terminated"}
  T8 = enum16{"USB6210", "USB6218AI", "USB6218AO", "LSI218", "LSI336"}
  T9 = cluster{"TimeArray":timestamp[], "Filtered X":dbl[]}[]
  T10 = cluster{"TimeArray (USB6218)":timestamp[], "DataArrayConv (USB6218)":dbl[]}[]
  T11 = cluster{"Label":string, "Active?":bool, "VISA resource name":refnum<visa-resource-name>, "Device":enum16{"Agilent34401A", "ADCMT7351", "HP3478A", "ADCMT7451"}, "Measurement":enum16{"DC Volts", "DC Currents", "2-Wire Resistance", "4-Wire Resistance"}, "FileFormat":string}[]
  T12 = enum16{"USB6210", "USB6218AI", "USB6218AO", "LSI218", "LSI336"}[]
  T13 = cluster{"Label":string, "Active?":bool, "Source":enum16{"USB6210", "USB6218AI", "USB6218AO", "LSI218", "LSI336"}, "SourceLabel":string, "FileFormat":string}[]